vi "Derivative of intensity graph-JKI SM.vi"() -> ()   [LabVIEW 2016] (continued)
  out "Linecut of Data 2":dbl[](graph)=[-2.8940890309223817e-07, -2.8218521036059675e-07, -2.750973803393701e-07, -2.681616119378308e-07, -2.61387573568958e-07, -2.5478180962496336e-07, -2.4834119759203e-07, -2.420613677656113e-07, -2.3594225731410755e-07, -2.2997972418850213e-07, -2.241723657896068e-07, -2.1854403296820515e-07, -2.1313554718359294e-07, -2.0796968419626724e-07, -2.030434637651495e-07, -1.983489854224866e-07, -1.9386884996078016e-07, -1.895787013930564e-07, -1.8547209206844587e-07, -1.8153372211331362e-07, -1.7771205918604306e-07, -1.739502529545922e-07, -1.702136181006313e-07, -1.6649310431306212e-07, -1.6280311122904338e-07, -1.5916752687039784e-07, -1.555998721568888e-07, -1.5209692914048345e-07, -1.486500041030232e-07, -1.4525555535832494e-07, -1.4191535498682274e-07, -1.3863768378600376e-07, -1.3543095716820107e-07, -1.322853298810876e-07, -1.291743587740751e-07, -1.260720429075625e-07, -1.2296223044263634e-07, -1.1984302292608645e-07, -1.1672013219342599e-07, -1.1359758377231182e-07, -1.1047856177345167e-07, -1.0736997066068235e-07, -1.0428240544729037e-07, -1.0122339033700634e-07, -9.819398582292763e-08, -9.519193566414333e-08, -9.220946170366257e-08, -8.92327373420117e-08, -8.625306684610114e-08, -8.327284300950467e-08, -8.029642598568983e-08, -7.73260760798728e-08, -7.436914388829862e-08, -7.14381264884156e-08, -6.854693712589017e-08, -6.570798514265498e-08, -6.292580108524908e-08, -6.019576814030563e-08, -5.751161009999894e-08, -5.487259825139198e-08, -5.228527113440777e-08, -4.975763820303616e-08, -4.728625682361953e-08, -4.486035757043568e-08, -4.247921749069906e-08, -4.0149036923674086e-08, -3.787148604762361e-08, -3.564475732299799e-08, -3.3472217300703734e-08, -3.136800219835929e-08, -2.9346409286532312e-08, -2.7400856454244e-08, -2.5511949128066436e-08, -2.367389206476488e-08, -2.1892905356020464e-08, -2.0175369344784737e-08, -1.852331987837496e-08, -1.69332269733478e-08, -1.5403565771935553e-08, -1.3943007872010564e-08, -1.2568050902960815e-08, -1.1294410331000255e-08, -1.012795554487589e-08, -9.061368130225111e-09, -8.078062620749276e-09, -7.157081015326442e-09, -6.279300001228574e-09, -5.42984791426857e-09, -4.603079184239391e-09, -3.808425672035557e-09, -3.0610262586367096e-09, -2.3732419642355494e-09, -1.7568424473291757e-09, -1.2279142641711952e-09, -8.002906467767922e-10, -4.76079301960497e-10, -2.4962039525342024e-10, -1.0875602227448447e-10, -3.548647834761396e-11, -8.224269538710525e-12, -5.828653148722821e-12, -1.4846612653496764e-11, -2.738889042657504e-11, -3.6902045319663076e-11, -4.1097623875271417e-11, -4.248733339086027e-11, -4.225480190923523e-11, -4.0073979006824705e-11, -3.6450390311194335e-11, -3.055163578303337e-11, -2.4351717257005638e-11, -2.102900179997745e-11, -1.850002706577997e-11, -1.5690568476919607e-11, -1.6638405929517314e-11, -2.282297995662489e-11, -2.8991982502704996e-11, -2.87729861305321e-11, -2.082041253168646e-11, -1.0950241327472767e-11, -5.94590536548409e-12, -6.124986382954428e-12, -7.1494587646023375e-12, -4.928026294178966e-12, -5.039119727047793e-13, 1.1691591478772948e-12, -1.9107212913616455e-12, -6.255112260036383e-12, -9.008420954114937e-12, -1.3057481266026498e-11, -1.928250493153049e-11, -2.298425366524667e-11, -2.198191289466519e-11, -1.893309421987613e-11, -1.6154553087490094e-11, -1.437079321309192e-11, -1.344083346264782e-11, -1.25929559540578e-11, -1.2579885553627824e-11, -1.4669539311777593e-11, -1.8112306643604654e-11, -2.165514312346446e-11, -2.394006737361059e-11, -2.2851467540324384e-11, -1.878226695129277e-11, -1.3811404313493993e-11, -1.1519665109555765e-11, -1.549763142709065e-11, -2.349514060223467e-11, -3.080966794426603e-11, -3.485149317671265e-11, -3.608941151608546e-11, -3.619185944432123e-11, -3.502236210343212e-11, -3.1615411305625565e-11, -2.5483220841765845e-11, -1.860920101705543e-11, -1.43390039557708e-11, -1.29379357541215e-11, -1.1376484518041533e-11, -8.09133430449214e-12, -5.667619055232239e-12, -6.1606356706996954e-12, -7.629299546284907e-12, -9.142578886729198e-12, -1.2541839225768736e-11, -1.6107589087197174e-11, -1.6173498693157964e-11, -1.4077592615147258e-11, -1.518305240939637e-11, -2.035050738432652e-11, -2.295880275862534e-11, -1.8657566141032195e-11, -1.059853736797566e-11, -3.798502170809853e-12, -1.6860676523363e-12, -3.731534128144562e-12, -4.780030058625379e-12, -2.953548312715921e-12, -2.0423521748336577e-13, 2.597419598843827e-12, 5.205097768140681e-12, 8.484894768670406e-12, 1.3363134206746872e-11, 1.7286172829092162e-11, 1.611370764411294e-11, 1.0617642545926209e-11, 6.726903431021291e-12, 6.989814545592153e-12, 7.72669496087859e-12, 7.729326538141858e-12, 8.992020683980025e-12, 9.614090082740139e-12, 5.538178504236205e-12, -2.4224000094075435e-12, -1.1199084476206675e-11, -1.9756326765894443e-11, -2.3129603963462973e-11, -1.7521481175240465e-11, -9.197721382017598e-12, -4.776965598906869e-12, -3.179260883441297e-12, -1.3916368059277791e-12, -7.962454600779184e-13, -6.206423007224318e-12, -1.7810691469904432e-11, -2.951467755447288e-11, -3.728176581369654e-11, -3.905209374276768e-11, -3.463346173233956e-11, -2.993298165578e-11, -3.0955271243153805e-11, -3.6257328722476964e-11, -4.0229887318282316e-11, -4.108144684148246e-11, -3.974737801554388e-11, -3.7165388792950676e-11, -3.442799948560981e-11, -3.1926419211695314e-11, -3.094731026192446e-11, -3.269173836301527e-11, -3.679349357346085e-11, -4.237634643149402e-11, -4.7032441280388325e-11, -4.575218770719866e-11, -3.6511856303236086e-11, -2.453988175102419e-11, -1.5897511837341424e-11, -1.2194798965793157e-11, -1.2769908868928286e-11, -1.583302795592875e-11, -1.839105762878466e-11, -1.8658147954917888e-11, -1.766589457325361e-11, -1.8424031653456276e-11, -2.0939825746159386e-11, -2.2491574009841726e-11, -2.37161727600735e-11, -2.5378023790577324e-11, -2.4667736899308864e-11, -2.0213779092230966e-11, -1.5835775062234915e-11, -1.4094415987625756e-11, -1.1705374447692051e-11, -6.584910528214012e-12, -1.6040906320380515e-12, -4.660119006047347e-13, -2.492740933819355e-12, -4.700548030424815e-12, -5.8724581410409235e-12, -4.660384107828449e-12, -1.9330184698207363e-12, 4.932451167041682e-13, 5.40180087507143e-12, 1.2661572193603058e-11, 1.6282136325177016e-11, 1.5141289778632374e-11, 1.0397445916458606e-11, 1.301372381251656e-12, -8.433865220774808e-12, -1.2557648021047707e-11, -7.848707930840445e-12, 2.230065100626399e-12, 1.0210390442654216e-11, 1.2545688629683348e-11, 9.962579622791734e-12, 5.327757730688172e-12, 3.792011893100133e-12, 6.289396601785914e-12, 6.9361476270789625e-12, 1.6921866018368433e-12, -7.480137026141833e-12, -1.5379633265526467e-11, -1.7767869850836955e-11, -1.2443322645761812e-11, -9.660600689856979e-13, 8.848092517460705e-12, 9.06580116766827e-12, 8.959421935900045e-13, -7.27954898668913e-12, -1.0168202143694001e-11, -8.054358681203483e-12, -5.393059291965451e-12, -4.940288505933282e-12, -4.256285747744637e-12, -3.826675690178256e-12, -7.336960432702211e-12, -1.309672008956676e-11, -1.5669009477628147e-11, -1.3923783740630542e-11, -1.0447604241746778e-11, -8.262840777791794e-12, -8.80904332033168e-12, -9.871140272746366e-12, -6.981729815805452e-12, -4.245141487077308e-13, 3.735125146795945e-12, 2.0637194223815546e-12, -2.8161392954633543e-12, -5.4596713685967705e-12, -3.1864472235988506e-12, 3.2239404165871712e-12, 1.0553363854420847e-11, 1.540723978620603e-11, 1.7954956438135358e-11, 1.838011179584692e-11, 1.551304741351347e-11, 1.0566601419640193e-11, 6.999161549293734e-12, 5.669197578119697e-12, 4.223135106888298e-12, 2.9158946822266156e-12, 4.815850189157709e-12, 9.446968260816934e-12, 1.2773501660927206e-11, 1.4702074749967083e-11, 1.7243285250520527e-11, 1.8900359902979115e-11, 2.0012350654596968e-11, 2.192158937545363e-11, 2.2119051943997926e-11, 1.9153588619723156e-11, 1.3457588259123014e-11, 7.929745223933709e-12, 7.764453322899451e-12, 1.1427659261215268e-11, 1.2218189840188382e-11, 1.0655993297653498e-11, 1.1938846745131875e-11, 1.3649496720017005e-11, 8.78154225263354e-12, -1.7224904349426275e-12, -9.385802439437218e-12, -8.951834758772276e-12, -2.438006974566303e-12, 3.060726442911228e-12, 2.728002108970522e-12, 1.2030435125714478e-12, 3.017569437970258e-12, 6.509335598467289e-12, 1.1041829064489001e-11, 1.3903680182577143e-11, 1.0313296014627426e-11, 7.243543751496639e-13, -9.10314875213029e-12, -1.5938815837317135e-11, -2.0921981047208584e-11, -2.1831491976361788e-11, -1.7012379815334596e-11, -1.2254005782942568e-11, -1.3210155299076422e-11, -1.7506934368553036e-11, -2.175636653207547e-11, -2.3987802293481042e-11, -2.1993305750057686e-11, -1.7590983642691515e-11, -1.1825032153325605e-11, -3.402913616444025e-12, 5.788513515495702e-12, 1.06051651945475e-11, 9.404669779143716e-12, 5.497486034493784e-12, 1.7815057046293091e-12, -4.968923486050722e-13, -1.3827354208238276e-12, -1.8234281451874533e-12, -1.7834522419839544e-12, 1.1650405969782519e-12, 8.282071952119584e-12, 1.6292996232852066e-11, 2.157689586678857e-11, 2.317778580608355e-11, 1.9927485421310814e-11, 1.2722650592904814e-11, 7.806483907218675e-12, 8.524528481987509e-12, 9.2513353928138e-12, 6.562550106740226e-12, 5.681317119375169e-12, 8.250614275667403e-12, 8.84923432218704e-12, 6.7373192175309534e-12, 5.1824832839794735e-12, 4.989144693078373e-12, 6.408081941629998e-12, 9.857940608712214e-12, 1.3666683587227867e-11, 1.4192872984893849e-11, 1.0552017135482878e-11, 4.673078366449931e-12, -1.9484245738993034e-12, -7.655629000441798e-12, -1.0301189009849796e-11, -8.540618207565813e-12, -4.1075734679155616e-12, -1.0961114439081418e-12, -2.529136826690413e-12, -8.735009934911757e-12, -1.551636362325879e-11, -1.971380080512105e-11, -2.4172273238734502e-11, -2.7859728832145033e-11, -2.587927069308313e-11, -1.9398004400440322e-11, -1.0531701328024916e-11, -1.5283667588723417e-12, 1.7519995256613797e-12, -1.0822948167828526e-12, -6.5596295255879636e-12, -1.372892015732692e-11, -2.0647593371330244e-11, -2.4572497789778387e-11, -2.3246448676992856e-11, -1.724349543084394e-11, -1.148906589082513e-11, -8.724906258309504e-12, -8.875472111849136e-12, -1.156812831686916e-11, -1.401147984500808e-11, -1.4421209797338631e-11, -1.3194325901493864e-11, -8.921073456720071e-12, -1.7079767247970636e-12, 5.153878890642483e-12, 8.277394835914015e-12, 5.200606434891234e-12, -3.0955990464275993e-12, -1.15113274549941e-11, -1.35989015012078e-11, -8.372393228296754e-12, -1.950060410278727e-12, 1.0397950884352703e-12, 2.05392326011597e-12, 3.9368531072437086e-12, 6.21709086108692e-12, 7.791793620762215e-12, 7.022918645137944e-12, 1.3173879416276409e-12, -6.901762657147866e-12, -1.2186251566125642e-11, -1.028804134906533e-11, 1.335660591492371e-12, 1.7493132275063488e-11, 2.6432766278136314e-11, 2.2936983581043868e-11, 1.2333121148947708e-11, 1.967680724456929e-12, -4.568015513852521e-12, -7.0854550896304396e-12, -4.982658034195635e-12, 9.075238906641379e-13, 5.398693347958892e-12, 4.591360398658498e-12, -1.5292556569915973e-12, -8.973667999151151e-12, -1.358273041572405e-11, -1.463979440466434e-11, -1.1523275601378697e-11, -6.151642015222169e-12, -1.6354052134162272e-12, 2.1419399426594397e-12, 5.020994579161354e-12, 7.191050722557544e-12, 7.948899252258628e-12, 4.2829830986390974e-12, -1.294295828499559e-12, -3.555625192562257e-12, -3.545539614611422e-12, -2.931106129713205e-12, -1.4701197266862009e-12, -2.2552433482491134e-13, 1.3440762578271492e-12, 4.143699467909959e-12, 7.789119340212557e-12, 9.5604198325248e-12, 4.403165132258261e-12, -8.452730171787493e-12, -2.300129192112561e-11, -3.2682922071540167e-11, -3.6497155413923733e-11, -3.72797326969456e-11, -3.657425284550991e-11, -3.46819897249427e-11, -3.0045010167691964e-11, -2.0542115734408094e-11, -1.0189703586248629e-11, -5.204221322687156e-12, -2.8258242631179308e-12, 2.43087927815717e-12, 8.074031430373864e-12, 8.151958100494352e-12, 2.0911425182147365e-13, -1.0675229042665783e-11, -1.597182369834803e-11, -1.5237703854225867e-11, -1.3610760910223127e-11, -1.05920862076095e-11, -4.672946687357804e-12, 1.5520500681798366e-12, 5.893095225456349e-12, 8.221564571007633e-12, 7.813171632672606e-12, 2.615369752659338e-12, -4.83533254989336e-12, -9.533734936158468e-12, -1.156761015308507e-11, -9.765904333603256e-12, -8.213035706642914e-13, 1.0813545175760329e-11, 1.6598926489665836e-11, 1.3647075999837657e-11, 6.93137347610472e-12, 4.199305462600087e-12, 7.408890903443559e-12, 1.099731812604974e-11, 1.0061292448833692e-11, 6.721831796966581e-12, 4.90601561249371e-12, 3.020311018028335e-12, -1.0046080106881757e-12, -4.387943169564147e-12, -4.457516375801223e-12, -4.2586573551127085e-13, 6.327900570456704e-12, 1.1880832983464011e-11, 1.144108081630853e-11, 4.1071509874510135e-12, -3.655210471444279e-12, -7.9869662184049e-12, -1.1056061401165982e-11, -1.2820322075315447e-11, -1.0721883688907626e-11, -5.262026729864167e-12, 3.093178667611112e-13, 4.226345170367926e-12, 6.2573554049032985e-12, 5.3280044322146726e-12, 1.3930654468456938e-12, -2.1359929319086752e-12, -5.0220789073138604e-12, -8.55503372676558e-12, -9.41830424268446e-12, -7.954872687236778e-12, -9.441372267032215e-12, -1.4687903762317724e-11, -2.1679329697375027e-11, -3.029542836365849e-11, -3.674245597786376e-11, -3.461055957500759e-11, -2.588253785010316e-11, -1.6347982489750724e-11, -6.707305352681958e-12, 1.1197136024465752e-12, 4.147210090800868e-12, 3.4865653210524286e-12, 4.581963028969805e-13, -5.4131945101485526e-12, -1.1878402094227307e-11, -1.3595758522327208e-11, -9.336139437172209e-12, -4.495985840536723e-12, -3.665546789669109e-12, -5.286542474984242e-12, -6.820966486594253e-12, -9.336004078294232e-12, -1.2804170330517656e-11, -1.464292363961387e-11, -1.4079621041501848e-11, -1.0521645337367027e-11, -4.220886275725529e-12, -5.222842467256578e-13, -2.8754261673526258e-12, -7.26345478741605e-12, -9.711847471466374e-12, -7.914472823869381e-12, -6.917980577121753e-13, 6.274899868417e-12, 7.276559562505807e-12, 2.646688866639234e-12, -4.158445754327833e-12, -8.690351479361557e-12, -1.030455386535592e-11, -9.528627945815406e-12, -6.735760013664561e-12, -5.5167424274532755e-12, -6.382482605769598e-12, -5.980772930811475e-12, -3.6003759581356943e-12, 4.4848746838119396e-13, 5.924501953616253e-12, 1.0200599545872995e-11, 1.2433441659682734e-11, 1.568695115733552e-11, 1.8960718442839018e-11, 1.7907555957967235e-11, 1.4227170632246267e-11, 1.3983556287164174e-11, 2.0895003060661385e-11, 3.401912125320816e-11, 4.707575608781025e-11, 5.1934463431664506e-11, 4.6999595381039817e-11, 3.954417132343792e-11, 3.4407615250988635e-11, 2.675734036864282e-11, 1.458376645843035e-11, 5.9128168199653285e-12, 5.52190309628963e-12, 8.787979443888981e-12, 1.1321969588781433e-11, 1.3251461508416912e-11, 1.3978508227983467e-11, 1.2550854621223148e-11, 1.2494322957013047e-11, 1.622943311952701e-11, 2.1075004154421106e-11, 2.6292120730628217e-11, 3.052828348025271e-11, 3.072447762411743e-11, 2.8952098070404286e-11, 2.7074172816998376e-11, 2.3294502796967226e-11, 1.8815115494587002e-11, 1.8071757500876235e-11, 2.043801049674637e-11, 2.1453289442479065e-11, 2.1026649061994397e-11, 2.1594769542120247e-11, 2.1943447847138888e-11, 2.075973246346161e-11, 2.0756776392065918e-11, 2.3085625872079274e-11, 2.754776388726862e-11, 3.5570798336213526e-11, 4.376992926709734e-11, 4.59070609191288e-11, 4.30325569381393e-11, 3.9932853525421607e-11, 3.835848865680091e-11, 3.828358697769738e-11, 4.005574455222349e-11, 4.4419870003607725e-11, 4.989701363013777e-11, 5.41269047685357e-11, 5.675147184238193e-11, 5.680368381620014e-11, 5.532221705045306e-11, 5.754884153975605e-11, 6.109952829632858e-11, 5.825661270312156e-11, 5.044552901803984e-11, 4.269752996451563e-11, 3.554041743595204e-11, 2.8867347993227685e-11, 2.5281708777280754e-11, 2.4376693739590814e-11, 2.1796408594452015e-11, 1.908728339225866e-11, 2.038712584071296e-11, 2.3779444689366904e-11, 2.7997515842014546e-11, 3.410107357336413e-11, 3.857323029135071e-11, 3.9289885218313416e-11, 3.994755294409079e-11, 4.161764363436933e-11, 4.106816091913509e-11, 3.699802827256904e-11, 3.0430396249010847e-11, 2.1813066435916014e-11, 1.2271733075639863e-11, 4.9552086052936795e-12, 1.59925140174941e-12, 1.4703085717474907e-12, 4.106858390568611e-12, 6.741321490730638e-12, 5.4727740144327445e-12, 3.545629806506765e-12, 7.747011922142562e-12, 1.6802955916934067e-11, 2.4186088875518423e-11, 2.889927214572701e-11, 3.301859623309055e-11, 3.6048296250859264e-11, 3.828115368900597e-11, 4.0231035811191867e-11, 3.953546727782567e-11, 3.574865402639116e-11, 3.439662860502771e-11, 3.7663022746057616e-11, 4.049876653585271e-11, 4.141258455247492e-11, 4.2888476090115246e-11, 4.50309592793821e-11, 4.748081680828003e-11, 4.878624431148641e-11, 4.432111415585341e-11, 3.479442440212306e-11, 2.4738021489416685e-11, 1.8060032881750395e-11, 2.1698587655981554e-11, 3.435462268879638e-11, 4.553184895422111e-11, 4.9815167279958966e-11, 4.850763922201503e-11, 4.6548225926384655e-11, 4.6622063791712037e-11, 4.6542656050117435e-11, 4.50164724961238e-11, 4.3177710051180646e-11, 4.191583910728815e-11, 3.994843447265572e-11, 3.639611467329391e-11, 3.379010759353175e-11, 3.5087778931594356e-11, 3.9223341978458535e-11, 4.2460948790422444e-11, 4.3284578029637285e-11, 4.386213284717559e-11, 4.5682570972923595e-11, 4.576393572249709e-11, 4.1710708354234745e-11, 3.413911964016388e-11, 2.619818258422197e-11, 2.1315420232006122e-11, 1.8357757755338573e-11, 1.5651449669770567e-11, 1.4027050973119977e-11, 1.427292956314629e-11, 1.4595155367250777e-11, 1.3126437929700617e-11, 1.1041347517523253e-11, 1.0485001539546375e-11, 1.257249780459313e-11, 1.5067339003510168e-11, 1.34144952514772e-11, 6.382342874520162e-12, -1.4879070113428431e-12, -6.251910202181846e-12, -7.818858224837596e-12, -6.727824029861449e-12, -3.0602951827382167e-12, 4.355700938375553e-12, 1.428689152472854e-11, 2.0752196678066787e-11, 1.9782977657157478e-11, 1.5586715575282498e-11, 1.3873304280412231e-11, 1.4765999841124256e-11, 1.6118557458355362e-11, 1.5713054965656394e-11, 1.4449661896940338e-11, 1.4158386655358312e-11, 1.476657074995396e-11, 1.4939874784825935e-11, 1.1835441542004752e-11, 8.902172518610685e-12, 1.0982271193334465e-11, 1.393492135209244e-11, 1.3329688624610254e-11, 1.2226425380543165e-11, 1.4419287900511152e-11, 1.868434226699991e-11, 2.21263513229607e-11, 2.3721373913650488e-11, 2.458766255048655e-11, 2.520545979216694e-11, 2.5445912224478432e-11, 2.6902444653042622e-11, 3.0902782077385675e-11, 3.59227691898179e-11, 3.728193119839106e-11, 3.320949219589552e-11, 2.8540428949919275e-11, 2.7682058948402316e-11, 3.061815980053606e-11, 3.4843335706753997e-11, 3.7735881223672336e-11, 3.796283254423637e-11, 3.5674102018748767e-11, 3.237322198913811e-11, 2.8585234575028694e-11, 2.524952964620034e-11, 2.7501470297456414e-11, 3.8254585130472957e-11, 4.961558102652725e-11, 5.090215003579e-11, 4.3531583093345775e-11, 3.533257809265555e-11, 2.7935847096028427e-11, 1.9306056973678287e-11, 1.0620382878490663e-11, 6.397594998773019e-12, 8.411378409736194e-12, 1.4922861585990827e-11, 2.223971632224944e-11, 2.586141168526224e-11, 2.701867275577852e-11, 3.023474668302981e-11, 3.218056844296344e-11, 2.776238336099858e-11, 2.0224587066257995e-11, 1.3814298857960018e-11, 9.618150383115673e-12, 8.212004353315733e-12, 8.063623963360287e-12, 7.01233091521858e-12, 6.577624554284749e-12, 8.758831452154896e-12, 1.2156076928679522e-11, 1.6155808913971643e-11, 2.1861559865862723e-11, 2.6191664021971177e-11, 2.483772302904293e-11, 2.1108574426577516e-11, 2.1778894335452237e-11, 2.6945196370807634e-11, 3.0691737915303356e-11, 2.8969768035365254e-11, 2.3160061740501135e-11, 1.7923447667542103e-11, 1.5550581527512263e-11, 1.6557638967519803e-11, 2.05127259246592e-11, 2.473838512186914e-11, 2.99889412574551e-11, 3.605131107559364e-11, 4.017096620083209e-11, 4.139172941100424e-11, 3.7386546115120144e-11, 2.8280657763484645e-11, 2.0594160937796013e-11, 1.9553535915506265e-11, 2.3654068278324007e-11, 2.7715172942157956e-11, 2.819763566326079e-11, 2.7409582362883298e-11, 2.8725428222488512e-11, 2.9728287772738024e-11, 2.5995741577426873e-11, 1.9427443001716098e-11, 1.565404155479251e-11, 1.5412962671600546e-11, 1.5016779000858612e-11, 1.0747430042492492e-11, 3.1768089326546723e-12, -2.9382906585806534e-12, -7.183997895918567e-12, -1.1476811053778265e-11, -1.3219479194740647e-11, -1.2091507924500355e-11, -1.2441404541913543e-11, -1.7006849520508685e-11, -2.4947724382139613e-11, -3.319466208802942e-11, -3.93936028751847e-11, -4.472739481372698e-11, -5.1437126190108995e-11, -5.743842547111449e-11, -5.951912983965276e-11, -5.84282649024997e-11, -5.7651164699486547e-11, -6.294110420321254e-11, -7.579253626647103e-11, -9.113308920152027e-11, -1.0732884452328227e-10, -1.2439000352790445e-10, -1.362577188283552e-10, -1.3860273054222297e-10, -1.360598040603649e-10, -1.3628565944569278e-10, -1.4339765738323208e-10, -1.5475811559588175e-10, -1.6421583392299495e-10, -1.70762138805023e-10, -1.7856145860556947e-10, -1.8743727163495584e-10, -1.9222020408524812e-10, -1.9192517612392896e-10, -1.9084685996537865e-10, -1.9188488794535773e-10, -1.962882044380347e-10, -2.0513286352946513e-10, -2.1599274998714897e-10, -2.259558102580132e-10, -2.3443064432784055e-10, -2.385613623527607e-10, -2.367963824806355e-10, -2.345932492000992e-10, -2.3506050407438354e-10, -2.3481936566710037e-10, -2.325454202130488e-10, -2.3182590380399555e-10, -2.3510172833986505e-10, -2.406051059213408e-10, -2.4754561225408115e-10, -2.557114102382339e-10, -2.6178555948565377e-10, -2.634120353438234e-10, -2.6169563706782656e-10, -2.588208417903325e-10, -2.572352623187533e-10, -2.5860585744264475e-10, -2.6302654261359033e-10, -2.684480244235243e-10, -2.734173835216019e-10, -2.789380728133596e-10, -2.854090599891106e-10, -2.9149897472272943e-10, -2.937159467923539e-10, -2.9086252075768506e-10, -2.869783721180875e-10, -2.8540142333855243e-10, -2.8496716791789273e-10, -2.835007028789644e-10, -2.822898973580844e-10, -2.83017986265416e-10, -2.844644297824711e-10, -2.84348616570163e-10, -2.8379079458794673e-10, -2.8718698853617357e-10, -2.954693663872105e-10, -3.0675710996263153e-10, -3.1863646716694584e-10, -3.2806967561770434e-10, -3.3263824768177325e-10, -3.293951646396497e-10, -3.211642312325179e-10, -3.1727822367687293e-10, -3.202584442036208e-10, -3.2636872425198945e-10, -3.322559166603789e-10, -3.354644486988945e-10, -3.3745164567437957e-10, -3.4069979308035874e-10, -3.440879059116009e-10, -3.4396230189896477e-10, -3.3655242302901894e-10, -3.242951754213375e-10, -3.147682035012691e-10, -3.09758950820402e-10, -3.0785179226964054e-10, -3.096660069800478e-10, -3.12367967066463e-10, -3.127048253696431e-10, -3.132840580338783e-10, -3.1547899818277355e-10, -3.16623439035482e-10, -3.145143429845095e-10, -3.0754357935502254e-10, -2.9747795727691977e-10, -2.8590730528816386e-10, -2.7152275958479235e-10, -2.5477848345951187e-10, -2.3710895269490615e-10, -2.2482316821560527e-10, -2.2527111941534628e-10, -2.348279616841208e-10, -2.451086125406314e-10, -2.513121013317493e-10, -2.5267111367255133e-10, -2.5181620104452924e-10, -2.51803778617962e-10, -2.532041420769055e-10, -2.544983553014328e-10, -2.5553304475359516e-10, -2.57370218129525e-10, -2.5859794587139265e-10, -2.566554453812346e-10, -2.544433305912939e-10, -2.5602253891728216e-10, -2.5893142382688945e-10, -2.5902965599023786e-10, -2.5690491715549246e-10, -2.562094910871496e-10, -2.5816074565491774e-10, -2.606272069569131e-10, -2.624755558768144e-10, -2.639450984111313e-10, -2.627893076019115e-10, -2.5963469172941667e-10, -2.6124225515409975e-10, -2.709234602427818e-10, -2.841033814685557e-10, -2.9489164062998424e-10, -3.0045941992561084e-10, -2.9879076769637797e-10, -2.907962500882942e-10, -2.823411374398335e-10, -2.7698805331488814e-10, -2.7198227295841446e-10, -2.66760437926745e-10, -2.6552840131225527e-10, -2.680240199079084e-10, -2.7200805579399774e-10, -2.786211360108172e-10, -2.874975975597856e-10, -2.9736720997177107e-10, -3.0846751376596147e-10, -3.198461357135976e-10, -3.29420109180591e-10, -3.3764930791726096e-10, -3.431728993006297e-10, -3.3833980080254576e-10, -3.2181979201869574e-10, -3.0276504894356323e-10, -2.890831327770462e-10, -2.821690200379822e-10, -2.7974895358874404e-10, -2.8025659694932375e-10, -2.825478373460058e-10, -2.852177697417637e-10, -2.8859506313646884e-10, -2.921223127326757e-10, -2.94492735649826e-10, -2.98009192505421e-10, -3.020035000764959e-10, -3.0183700045653746e-10, -2.9793810460720123e-10, -2.9429426662524416e-10, -2.9413556648775213e-10, -2.956745023385105e-10, -2.940724557473711e-10, -2.9052534819344446e-10, -2.8715147241825065e-10, -2.823246414505911e-10, -2.754858837792391e-10, -2.6718253181625536e-10, -2.6030522484316173e-10, -2.5862490253346696e-10, -2.6200988462061114e-10, -2.6699842542333255e-10, -2.6958645971402096e-10, -2.685018077764725e-10, -2.6625729908971983e-10, -2.6530298346105215e-10, -2.6583169110629015e-10, -2.6741479924643173e-10, -2.703537364690107e-10, -2.7590104418249973e-10, -2.813588852677852e-10, -2.809778990927319e-10, -2.7563212332163685e-10, -2.68204406658312e-10, -2.5930224884862044e-10, -2.541323759918927e-10, -2.565071086111615e-10, -2.6281131275256104e-10, -2.6924003221722695e-10, -2.764076416786395e-10, -2.848578924373651e-10, -2.9279086086396945e-10, -2.998637545795645e-10, -3.0505462427506586e-10, -3.045651669404588e-10, -2.9703145384598195e-10, -2.876118203027926e-10, -2.83521682006714e-10, -2.8404475709495946e-10, -2.835720116344828e-10, -2.8328617951377393e-10, -2.8752202689923624e-10, -2.941725255882044e-10, -2.978066878178572e-10, -2.9669767586963245e-10, -2.935166907228826e-10, -2.92093276406279e-10, -2.9379469041415784e-10, -2.957357413609668e-10, -2.9306893934226655e-10, -2.8541796084025373e-10, -2.780027609979395e-10, -2.740143235479234e-10, -2.7376899246638295e-10, -2.7731553749816434e-10, -2.8443289856345437e-10, -2.939582677780864e-10, -3.008013678819796e-10, -3.0147406597921476e-10, -2.995833913843125e-10, -2.9971300598578395e-10, -3.0039369556034337e-10, -2.989567566426567e-10, -2.9497999745290136e-10, -2.892287217221146e-10, -2.8390259171547476e-10, -2.7877776590975683e-10, -2.7603426201616866e-10, -2.791271366004494e-10, -2.841698296628249e-10, -2.8660340966299784e-10, -2.881488202794268e-10, -2.893428985122702e-10, -2.8548621596237926e-10, -2.7608428651157776e-10, -2.6912334390858275e-10, -2.691740779014742e-10, -2.7181312280019317e-10, -2.7459241171990615e-10, -2.7702932893009703e-10, -2.7513277851067665e-10, -2.698103607295403e-10, -2.6826058926418707e-10, -2.7332709079697383e-10, -2.825867063385152e-10, -2.9161281141068467e-10, -2.968102201997065e-10, -2.9838904630059864e-10, -2.961981692847394e-10, -2.890181887032996e-10, -2.779716163847304e-10, -2.6902787090068106e-10, -2.675802118937036e-10, -2.709589279469448e-10, -2.7605405068131046e-10, -2.8376961072576854e-10, -2.921252287581268e-10, -2.973398881585562e-10, -2.985540604747546e-10, -2.956595533203178e-10, -2.889510916468132e-10, -2.815692280302651e-10, -2.786347624480804e-10, -2.804576333046588e-10, -2.82067832676929e-10, -2.834482064586615e-10, -2.862239141194915e-10, -2.845419191359875e-10, -2.731393231490222e-10, -2.5568316078173645e-10, -2.3842288432592806e-10, -2.2492800466855273e-10, -2.147787442285775e-10, -2.0411464498598006e-10, -1.9179887817562718e-10, -1.818001367399064e-10, -1.757290981404682e-10, -1.6853104638359517e-10, -1.599174210482408e-10, -1.555228913223865e-10, -1.5725342048961687e-10, -1.644846968183484e-10, -1.7460384911444947e-10, -1.8360433580515635e-10, -1.879789981926387e-10, -1.8840551443323492e-10, -1.888353771339315e-10, -1.8969099741263147e-10, -1.9024993301903443e-10, -1.8931500129711534e-10, -1.8430941423007118e-10, -1.7715590731609578e-10, -1.7564851705199378e-10, -1.8319763734700583e-10, -1.9361175575038266e-10, -1.9991293509225652e-10, -2.0044485911887886e-10, -1.9658904079170522e-10, -1.8867566304683285e-10, -1.7891485017919798e-10, -1.7174345019962715e-10, -1.6798917713424406e-10, -1.6656312355990725e-10, -1.6573279220177242e-10, -1.6277867838515427e-10, -1.5731013759656216e-10, -1.4647503948215146e-10, -1.1515324415920093e-10, -3.935080270413761e-11, 1.0344393801415088e-10, 3.2823653907287383e-10, 6.421159963701627e-10, 1.0508239672753578e-09, 1.556502762883994e-09, 2.1493008879857615e-09, 2.816177560694013e-09, 3.557508239050816e-09, 4.390440211230907e-09, 5.334481075630683e-09, 6.392878597346859e-09, 7.554845937836172e-09, 8.809656652911219e-09, 1.0154989715608278e-08, 1.1605220105232825e-08, 1.3179567140700973e-08, 1.4876194019264124e-08, 1.6674253944853294e-08, 1.8560111759052268e-08, 2.0540373673269138e-08, 2.262439839505953e-08, 2.4881076757816235e-08, 2.7502869161575475e-08, 3.061853211700037e-08, 3.4117635970112586e-08, 3.7782000167305955e-08, 4.1452245541307266e-08, 4.506809424634262e-08, 4.8632601983748894e-08, 5.2159694231260575e-08, 5.5676276468474306e-08, 5.922009250753216e-08, 6.280219104068659e-08, 6.638239838347632e-08, 6.991240368594546e-08, 7.342984606051368e-08, 7.70513629322336e-08, 8.087498564831669e-08, 8.495038023629491e-08, 8.932244119554336e-08, 9.40443381277796e-08, 9.913973458546139e-08, 1.0457997230794205e-07, 1.1030367800555867e-07, 1.1624949463803816e-07, 1.2237541810843132e-07, 1.286724983937204e-07, 1.3516371272689553e-07, 1.418727945202124e-07, 1.487961715792217e-07, 1.5591070767854713e-07, 1.6320478329567495e-07, 1.706949985460585e-07, 1.7839988526093034e-07, 1.8630026359559254e-07, 1.9434867222524683e-07, 2.0250798012300995e-07, 2.1077071743172693e-07, 2.192333041900014e-07, 2.2847810270536458e-07]
  in  "Start viewing ?":bool
  in  "Wait between index":u32=10
  in  "stop viewing ?":bool
  in  "Pause viewing ?":bool
  in  "Decimate index":i32=1
  out "Linecut of derivative 2":cluster{dbl[], dbl[]}(graph)
  out "Y value":string="VsgL (V)= 0.0"
  out "Signal offset":string="= 871.361pA"
  in  "Multiplier":dbl=1.0
  in  "Input Data":dbl[][](graph)=array1229x321[394509 elements]
  in  "Step for derivative":dbl=15.0
  in  "Signal offset to Subtract":T3
  in  "Name":T4={"X"="Vsd (V)", "Y"="VsgL (V)", "Z"="I (A)", "dZ/dX"="dI/dV (S)"}
  in  "Remove signal offset ?":bool=TRUE
  in  "Cursor.Visible ? - Data":bool=TRUE
  in  "Cursor.Visible ? - Derivative":bool=TRUE
  in  "OK":bool
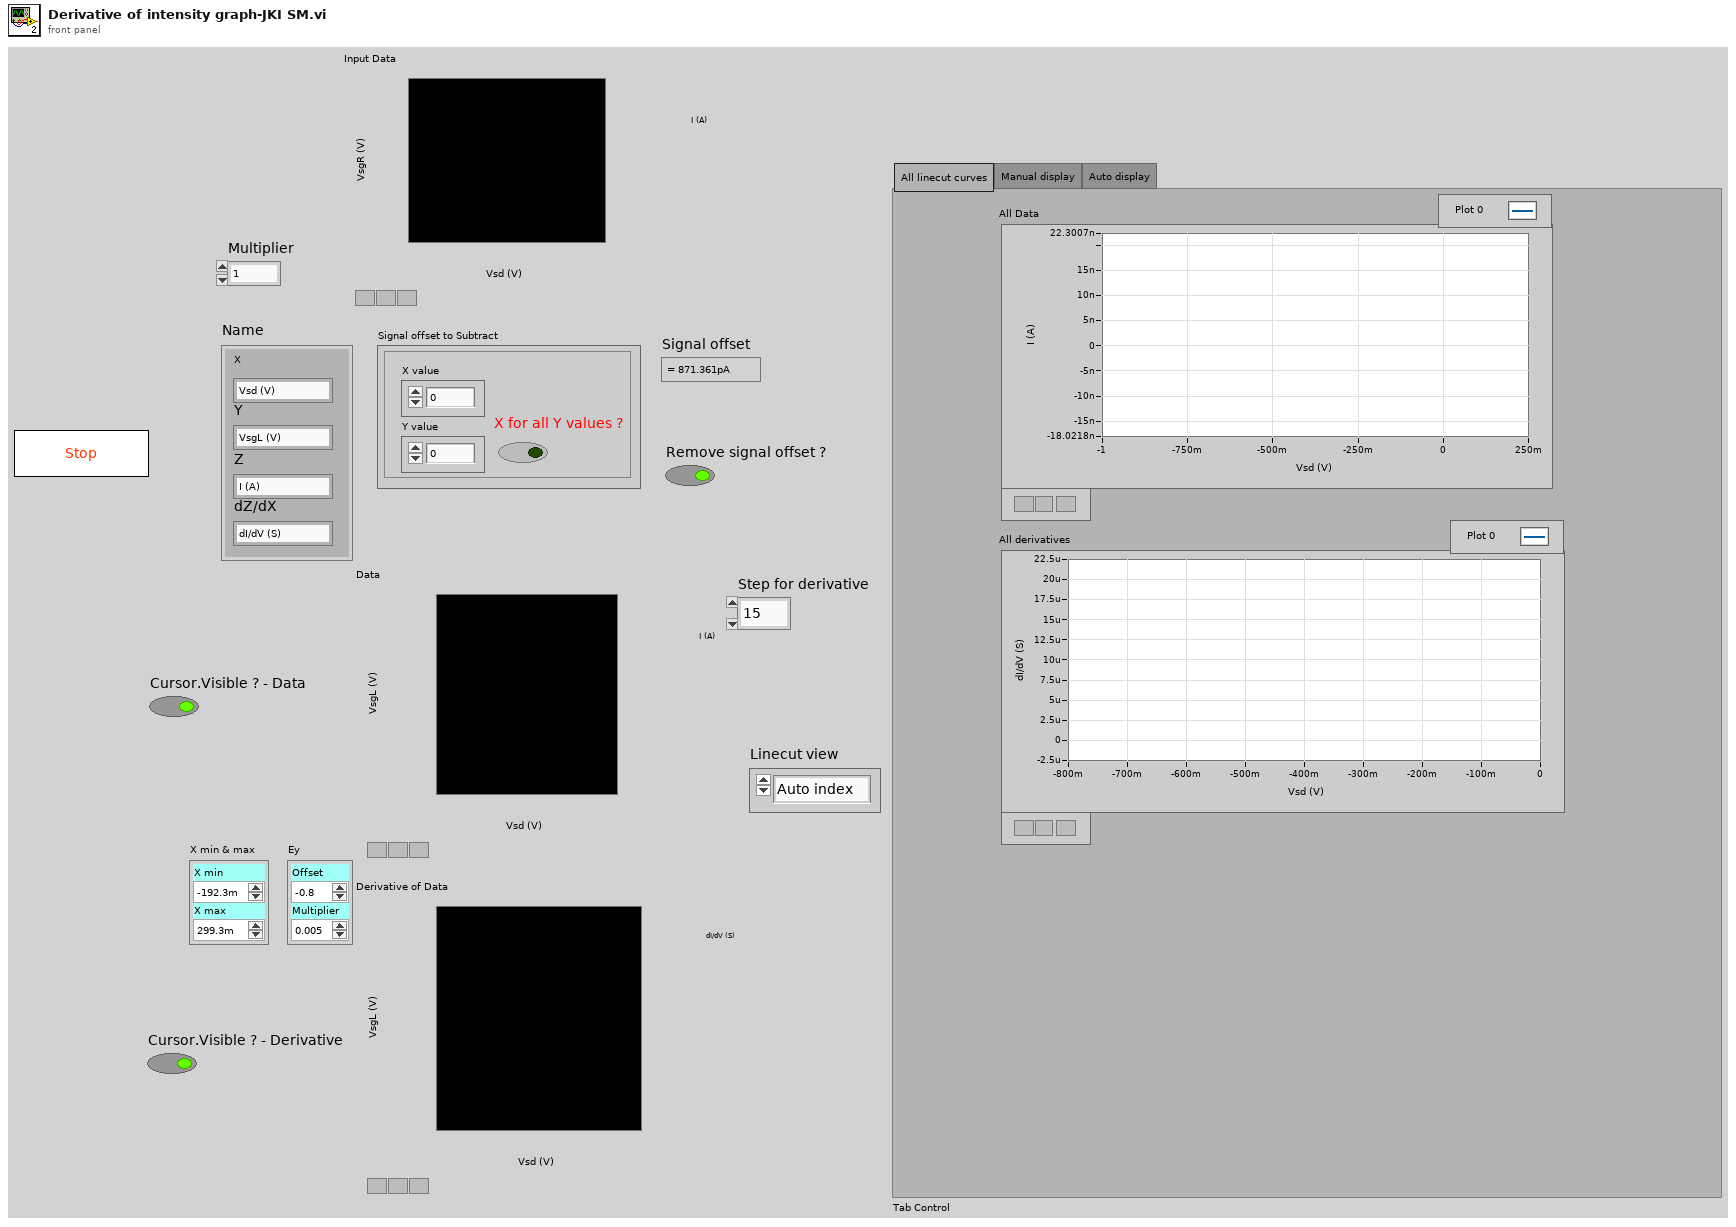
[diagram p1: front panel]
types:
  T1 = typedef "LVOffsetAndMultiplierTypeDef.ctl" = cluster{"Offset":dbl, "Multiplier":dbl}
  T2 = enum32{"All linecut curves", "Manual display", "Auto display"}
  T3 = cluster{"X value":dbl, "Y value":dbl, "X for all Y values ?":bool}
  T4 = cluster{"X":string, "Y":string, "Z":string, "dZ/dX":string}
  T5 = enum32{"Invalid", "Standard", "Closed", "Hidden", "Minimized", "Maximized"}
  T6 = enum32{"invalid app kind", "Development System", "Run Time System", "Student Edition", "Embedded LabVIEW", "Evaluation", "Custom"}
  T7 = cluster{"Core":cluster{"Current VI Reference":refnum<vi>, "Close Panel on Exit?":bool}, "Remove signal offset ?":bool, "Cursor.Visible?":bool, "Cursor.Visible? 2":bool, "Name":cluster{"X":string, "Y":string, "Z":string, "dZ/dX":string}, "Linecut view":enum16{"Manual index", "Auto index"}, "Signal offset to Subtract":cluster{"X value":dbl, "Y value":dbl, "X for all Y values ?":bool}, "Input Data":dbl[][], "Data":dbl[][], "X array":dbl[], "Step for derivative":dbl, "X min & max":cluster{"X min":dbl, "X max":dbl}, "Ey":T1, "Ex":T1, "All derivatives":cluster{dbl[], dbl[]}[], "Cursor X index":i32, "Cursor Y index":i32}
  T8 = cluster{"Current VI Reference":refnum<vi>, "Close Panel on Exit?":bool}
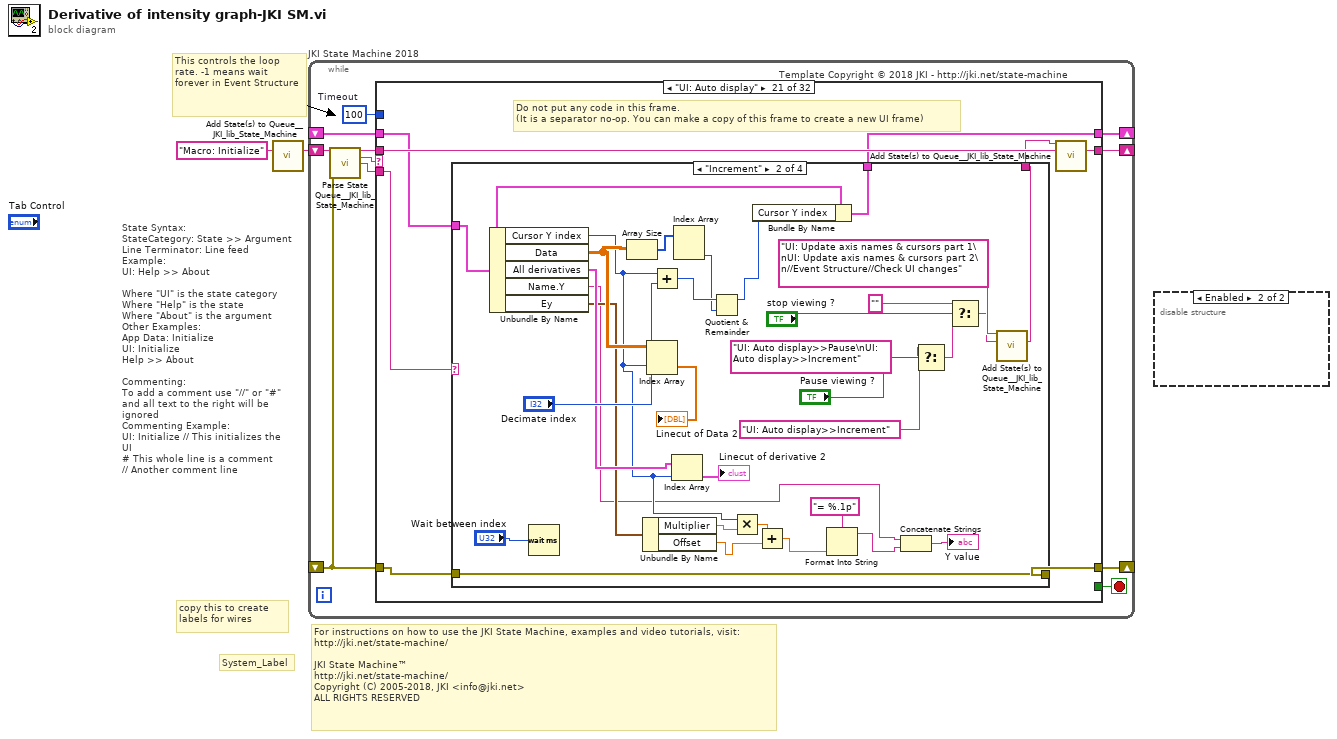
[diagram p0: block diagram]
diagram:
  # "For instructions on how to use the JKI State Machine, examples and video tutorials, visit:\nhttp://jki.net/state-machine/\n\nJKI State Machine™\nhttp://jki.net/state-machine/\nCopyright (C) 2005-2018, JKI <info@jki.net>\nALL RIGHTS RESERVED"
  # "State Syntax:\nStateCategory: State >> Argument\nLine Terminator: Line feed\nExample:\nUI: Help >> About\n\nWhere \"UI\" is the state category\nWhere \"Help\" is the state\nWhere \"About\" is the argument\nOther Examples:\nApp Data: Initialize\nUI: Initialize\nHelp >> About\n\nCommenting:\nTo add a comment use \"//\" or \"#\" and all text to the right will be ignored\nCommenting Example:\nUI: Initialize // This initializes the UI\n# This whole line is a comment\n// Another comment line"
  # "copy this to create labels for wires"
  # "This controls the loop rate. -1 means wait forever in Event Structure"
  # "System_Label"
  n1 = call <vilib>:"Add State(s) to Queue__JKI_lib_State_Machine.vi"("State(s) in (\"\")"="Macro: Initialize") -> ("States Out"=w2:string)  [unwired: 14 in]
  n2 = while "JKI State Machine 2018" {
    shift-right: [w6] -> _
    shift-left: _ -> [w5]
    shift-right: [w9] -> _
    shift-left: _ -> [w3]
    shift-right: [w8] -> _
    shift-left: w2 -> [w10]
    stop <- w7 stop-if-true
    w4 = 100  # Timeout
    # "Template Copyright © 2018 JKI - http://jki.net/state-machine"
    n3 = call <vilib>:"Parse State Queue__JKI_lib_State_Machine.vi"("State Queue"=w10, "Error In (no error)"=w3) -> ("Remaining States"=w12:string, "Current State"=w13:string, "Arguments"=w11:string)  [unwired: 11 in]
    n4 = case shown="\"UI: Auto display\"" w13 {
      selector: w13 -> [_ _ w80 _ _ _ _ _ _ _ _ _ _ _ _ _ _ _ _ _ _ _ _ _ _ _ _ _ _ _ _ _]
      tunnel: w12 -> [w20 w79 w84 w103 w109 w114 w118 w139 w145 w149 w153 w159 w170 w246 w256 w274 w280 w308 w318 w332 w340 w387 w392 w397 w407 w411 w419 w436 w450 w468 w497 w505]
      tunnel: w11 -> [_ _ _ _ _ _ _ _ _ _ _ w154 w164 _ _ _ _ _ _ _ w336 _ _ _ _ _ _ _ _ _ _ _]
      tunnel: w5 -> [w18 w76 w82 w96 w106 w112 w115 _ w140 w146 w150 w157 w166 w244 w253 w263 w277 w305 w315 w325 w335 w384 w389 w394 w404 w408 w416 w432 w438 w459 w495 w502]
      tunnel: [w17 w77 w86 w100 errorcluster {"status"=FALSE, "code"=0, "source"=""} ("error out") w111 w116 w136 w141 w147 w151 w155 w167 w236 w254 w272 w278 w306 w316 w330 w337 w385 w390 w395 w405 w409 w417 w434 w448 w465 w489 w503] -> w9
      tunnel: w3 -> [w16 w77 w85 w100 w105 w111 w116 w136 w142 w147 w151 w156 w168 _ w254 w272 w278 w306 w316 w330 w338 w385 w390 w395 w405 w409 w417 w434 w448 w466 w490 w503]
      tunnel: [w19 w78 w83 w102 w108 w113 w117 w138 w144 w148 w152 w158 w169 w245 w255 w273 w279 w307 w317 w331 w339 w386 w391 w396 w406 w410 w418 w435 w449 w467 w496 w504] -> w8
      tunnel: [_ _ _ _ _ TRUE _ _ _ _ _ _ _ _ _ _ _ _ _ _ _ _ _ _ _ _ _ _ _ _ _ _] -> w7
      tunnel: [w15 w76 w82 w101 w106 w112 w115 w137 w140 w146 w150 w157 w166 w244 w253 w262 w276 w305 w315 w324 w334 w384 w389 w394 w404 w408 w415 w431 w437 w458 w495 w502] -> w6
      tunnel: w4 -> [w14 _ _ _ _ _ _ _ _ _ _ _ _ _ _ _ _ _ _ _ _ _ _ _ _ _ _ _ _ _ _ _]
      frame "", "Event Structure", "Idle" {
        # "executes when the state queue is empty"
        n5 = event shown="[5] \"Multiplier\": Value Change" {
          selector: _ -> [_ _ _ _ _ _ _ _ _ _ _]
          dyn-events: _ -> [_ _ _ _ _ _ _ _ _ _ _]
          timeout: w14 -> [_ _ _ _ _ _ _ _ _ _ _]
          tunnel: w20 -> [w24 w29 w34 w39 w44 w49 w54 w59 w64 w69 w75]
          tunnel: [w23 w28 w33 w38 w43 w48 w53 w58 w63 w68 w74] -> w19
          tunnel: w18 -> [w21 w26 w31 w36 w41 w46 w51 w56 w61 w66 w72]
          tunnel: [w22 w27 w32 w37 w42 w47 w52 w57 w62 w67 w73] -> w17
          tunnel: w16 -> [w22 w27 w32 w37 w42 w47 w52 w57 w62 w67 w73]
          tunnel: [w21 w26 w31 w36 w41 w46 w51 w56 w61 w66 w72] -> w15
          event Timeout {
            (unwired) "Exit" ("State(s) in Front (\"\")")
            (unwired) "" ("State(s) in Front (\"\")")
            # "Timeout Frame\n(this will only execute if the Event Structure timeout is >= 0)"
            n6 = event-data() -> ()  [unwired: 1 in, 1 out]
            n7 = call <vilib>:"Add State(s) to Queue__JKI_lib_State_Machine.vi"("State(s) in (\"\")"=w24) -> ("States Out"=w23:string)  [unwired: 14 in]
          }
          event "X min & max": Value Change {
            # "Timeout Frame\n(this will only execute if the Event Structure timeout is >= 0)"
            n8 = event-data() -> ()  [unwired: 1 in, 6 out]
            n9 = call <vilib>:"Add State(s) to Queue__JKI_lib_State_Machine.vi"("State(s) in Front (\"\")"="UI: Update X Y setting\nData process: Create X array\nData process: Plot Derivative\nData process: Plot all linecut curves\nUI: Update axis names & cursors part 1\nUI: Update axis names & cursors part 2" ("State(s) in Front (\"\")"), "State(s) in (\"\")"=w29) -> ("States Out"=w28:string)  [unwired: 13 in]
          }
          event Value Change {
            # "Timeout Frame\n(this will only execute if the Event Structure timeout is >= 0)"
            n10 = event-data() -> ()  [unwired: 1 in, 6 out]
            n11 = call <vilib>:"Add State(s) to Queue__JKI_lib_State_Machine.vi"("State(s) in Front (\"\")"="UI: Update X Y setting\nData process: Create X array\nData process: Plot Derivative\nData process: Plot all linecut curves\nUI: Update axis names & cursors part 1\nUI: Update axis names & cursors part 2" ("State(s) in Front (\"\")"), "State(s) in (\"\")"=w34) -> ("States Out"=w33:string)  [unwired: 13 in]
          }
          event "Start viewing ?": Value Change {
            (unwired) "" ("State(s) in Front (\"\")")
            # "Timeout Frame\n(this will only execute if the Event Structure timeout is >= 0)"
            n12 = event-data() -> ()  [unwired: 1 in, 6 out]
            n13 = call <vilib>:"Add State(s) to Queue__JKI_lib_State_Machine.vi"("State(s) in Front (\"\")"="UI: Auto display>>Start" ("State(s) in Front (\"\")"), "State(s) in (\"\")"=w39) -> ("States Out"=w38:string)  [unwired: 13 in]
          }
          event "Step for derivative": Value Change {
            # "Timeout Frame\n(this will only execute if the Event Structure timeout is >= 0)"
            n14 = event-data() -> ()  [unwired: 1 in, 6 out]
            n15 = call <vilib>:"Add State(s) to Queue__JKI_lib_State_Machine.vi"("State(s) in Front (\"\")"="Data process: Plot Derivative\nData process: Plot all linecut curves" ("State(s) in Front (\"\")"), "State(s) in (\"\")"=w44) -> ("States Out"=w43:string)  [unwired: 13 in]
          }
          event "Multiplier": Value Change {
            # "Timeout Frame\n(this will only execute if the Event Structure timeout is >= 0)"
            n16 = event-data() -> ()  [unwired: 1 in, 6 out]
            n17 = call <vilib>:"Add State(s) to Queue__JKI_lib_State_Machine.vi"("State(s) in Front (\"\")"="Macro: Plot Data" ("State(s) in Front (\"\")"), "State(s) in (\"\")"=w49) -> ("States Out"=w48:string)  [unwired: 13 in]
          }
          event "Remove signal offset ?": Value Change {
            # "Timeout Frame\n(this will only execute if the Event Structure timeout is >= 0)"
            n18 = event-data() -> ()  [unwired: 1 in, 6 out]
            n19 = call <vilib>:"Add State(s) to Queue__JKI_lib_State_Machine.vi"("State(s) in Front (\"\")"="Data process: Remove signal offset\nData process: Create X array\nData process: Plot Derivative\nData process: Plot all linecut curves" ("State(s) in Front (\"\")"), "State(s) in (\"\")"=w54) -> ("States Out"=w53:string)  [unwired: 13 in]
          }
          event "Name": Value Change {
            # "Timeout Frame\n(this will only execute if the Event Structure timeout is >= 0)"
            n20 = event-data() -> ()  [unwired: 1 in, 6 out]
            n21 = call <vilib>:"Add State(s) to Queue__JKI_lib_State_Machine.vi"("State(s) in Front (\"\")"="UI: Update axis name\nUI: Update axis names & cursors part 1\nUI: Update axis names & cursors part 2" ("State(s) in Front (\"\")"), "State(s) in (\"\")"=w59) -> ("States Out"=w58:string)  [unwired: 13 in]
          }
          event "Linecut view": Value Change {
            # "Timeout Frame\n(this will only execute if the Event Structure timeout is >= 0)"
            n22 = event-data() -> ()  [unwired: 1 in, 6 out]
            n23 = call <vilib>:"Add State(s) to Queue__JKI_lib_State_Machine.vi"("State(s) in Front (\"\")"="UI: Select display mode" ("State(s) in Front (\"\")"), "State(s) in (\"\")"=w64) -> ("States Out"=w63:string)  [unwired: 13 in]
          }
          event "OK": Value Change {
            # "Exit Button Value Change (pressed) Event\n(this executes Macro: Exit to terminate the VI)"
            n24 = event-data() -> ()  [unwired: 1 in, 1 out]
            n25 = call <vilib>:"Add State(s) to Queue__JKI_lib_State_Machine.vi"("State(s) in Front (\"\")"="Macro: Exit", "State(s) in (\"\")"=w69) -> ("States Out"=w68:string)  [unwired: 13 in]
          }
          event Panel Close? {
            # "Discard the event because we'll close the front panel ourselves in Macro: Exit"
            # "Close Panel button (pressed) Event\n(this executes Macro: Exit to terminate the VI)"
            n26 = event-data() -> ()  [unwired: 1 in, 1 out]
            n27 = event-data("Discard?"=TRUE) -> ()  [unwired: 1 in, 1 out]
            n28 = call <vilib>:"Add State(s) to Queue__JKI_lib_State_Machine.vi"("State(s) in Front (\"\")"="Macro: Exit", "State(s) in (\"\")"=w75) -> ("States Out"=w74:string)  [unwired: 13 in]
          }
        }
      }
      frame "---------- Core ----------" {
        # "Do not put any code in this frame.\n(it is a separator no-op)"
        n29 = call <vilib>:"Add State(s) to Queue__JKI_lib_State_Machine.vi"("State(s) in (\"\")"=w79) -> ("States Out"=w78:string)  [unwired: 14 in]
      }
      frame Default {
        w89 = 42 items=["No error", "Argument error", "Memory is full", "Out of zone", "End of file", "File already open", "Generic file I/O error", "File not found", "File permission error", "Disk is full", "Duplicate path", "Too many files open", "System feature not enabled", "Resource file not found", "Cannot add resource", "Resource not found", "Image not found", "Image memory error", "Pen does not exist", "Config type invalid", "Config token not found", "Config parse error", "Config memory error", "Bad external code format", "Bad external code offset", "External code not present", "Null window", "Destroy window error", "Null menu", "Print aborted", "Bad print record", "Print driver error", "Windows error during printing", "Memory error during printing", "Print dialog error", "Generic print error", "Invalid device refnum", "Device not found", "Device parameter error", "Device unit error", "Cannot open device", "Device call aborted", "Generic error", "Cancelled by user", "Object ID too low", "Object ID too high", "Object not in heap", "Unknown heap", "Unknown object (invalid DefProc)", "Unknown object (DefProc not in table)", "Message out of range", "Invalid (null) method", "Unknown message", "Manager call not supported", "Bad address", "Network operation in progress", "Network operation timed out", "Connection is busy", "Network attribute not supported", "Network error", "Address in use", "System out of memory", "Connection aborted", "Connection refused", "Not connected", "Already connected", "Connection closed", "Initialization error (interapplication manager)", "Bad occurrence", "Wait on unbound occurrence handler", "Occurrence queue overflow", "Datalog type conflict", "Unused", "Unrecognized type (interapplication manager)", "Memory corrupt", "Failed to make temporary DLL", "Old CIN version", "Drag socket not found", "Failed to load drop-object", "Failed to register OLE object", "Failed to release OLE object", "Format specifier type mismatch", "Unknown format specifier", "Too few format specifiers", "Too many format specifiers", "Scan failed", "Newer CIN version", "Error converting to variant", "Runtime menu error", "Password tampered", "Variant attribute not found", "Incompatible variant data type", "Event data is not available", "Event Store is not present", "Occurrence is not found", "Event Queue is not created", "Event info is not available", "Refnum passed is NULL", "Error retrieving Class GUID", "Error retrieving CoClass GUID", "Error retrieving TypeLib GUID.", "Bad built application magic bytes.", "Specific driver is different from the specific driver associated with the Logical Name.", "There is no session opened to the class driver.", "Max Error", "MAX - Error with config objects", "MAX - Error loading configuration", "MAX - Group not supported"]